vi "UHR-Fleezers Control (host) - 12.0(oscillate_test).vi"() -> ()   [LabVIEW 2014] (continued)
            n2508 = local read "Number of F/B Scans (AOD)"() -> (w4839:u16)
            n2509 = Sign(1:w4822) -> (0:w4821:dbl)
            n2510 = Compound Arithmetic op=MULTIPLY(w4822, "MCL Step Position Ratio", "MCL/AOM Scale Tweak") -> (w4826:dbl)
            n2511 = Negate(x=w4821) -> (-x=w4818:dbl)
            n2512 = Multiply(x=w4818, y="MCL Step Increment (V_int)") -> (x*y=w4820:dbl)
            n2513 = Divide(x=w4826, y="MCL X Cal (nm/V)") -> (x/y=w4832:dbl)
            n2514 = Multiply(x=32767.0 ("y"), y=w4832) -> (x*y=w4838:dbl)
            n2515 = local read "Total Counts (ticks)"() -> (w4823:u32)
            n2516 = local read "Cycles/step (AOD)"() -> (w4834:u64)
            n2517 = local read "Scan steps (AOD)"() -> (w4835:u64)
            n2518 = Divide(x=w4838, y=10.0) -> (x/y=w4831:dbl)
            n2519 = Divide(x=w4831, y="MCL Step Increment (V_int)") -> (x/y=w4829:dbl)
            n2520 = Absolute Value(x=w4829) -> (abs(x)=w4817:dbl)
            n2521 = Compound Arithmetic op=MULTIPLY(w4835, w4834, w4823) -> (w4830:u64)
            n2522 = local write "wait to reset values"(w4845) -> ()
            n2523 = local write "MCL Scanning"(w4845) -> ()
            n2524 = Divide(x=w4830, y=w4817) -> (x/y=w4827:dbl)
            "MCL Count" <- w4827
            n2525 = xnode "Read/Write Control"("FPGA VI Reference In"=w4844, "error in"=w4843, "Scan steps (MCL)"=w4817, "Number of scans (MCL)"=w4839, "Cycles per step (MCL)"=u64 1, "Scan freq.  increment (MCL)"=w4820, "1D or 2D Scan?"=w4840, "MCL Scan Axis"=w4840, "Cont. Scan (MCL)"=w4840, "MCL count"=w4827) -> ("FPGA VI Reference Out"=w4842:T22, "error out"=w4841:errorcluster)
            n2526 = xnode "Read/Write Control"("FPGA VI Reference In"=w4842, "error in"=w4841, "AI to FIFO"=w4845, "APD to FIFO"=w4845, "Start scan"=w4845, "Start scan (MCL)"=w4845) -> ("FPGA VI Reference Out"=w4847:T22, "error out"=w4846:errorcluster)
          }
        }
        "Raster Scanning..." <- TRUE ("Scanning...")
      }
    }
    n2527 = local read "Flushing P3"() -> (w3622:bool)
    n2528 = case "Keep track of when Harvard Pump 3 is done flushing" shown="True" w3622 {
      frame False {
      }
      frame True {
        n2529 = local read "Flush rate (uL/m) P3"() -> (w4005:dbl)
        n2530 = local read "DMA Update Period (s)"() -> (w3999:dbl)
        n2531 = local read "HP3 Flush Time (s)"() -> (w4013:dbl)
        n2532 = Divide(x=w4005, y=60.0) -> (x/y=w4000:dbl)
        n2533 = feedback #6(0) -> (w4011:i32)
        n2534 = Increment(x=w4011) -> (x+1=w4006:i32)
        n2535 = Divide(x=w4013, y=w3999) -> (x/y=w4007:dbl)
        n2536 = Multiply(x=w3999, y=w4000) -> (x*y=w3998:dbl)
        n2537 = Greater?(x=w4006, y=w4007) -> (0:w4010:bool)
        n2538 = feedback #7(0.0) -> (w4001:dbl)
        n2539 = Compound Arithmetic op=MULTIPLY(w3999, w4006, w4000) -> (→"P3 Flush Volume (uL)":dbl)
        n2540 = case shown="True" w4010 {
          tunnel: w4006 -> [w4014 _]
          tunnel: [w4014 0] -> w4009
          frame False {
          }
          frame True {
            w4015 = FALSE ("Flushing P3")
            n2541 = local write "Inject Pump 3"(w4015) -> ()
            n2542 = local write "Flushing P3"(w4015) -> ()
            n2543 = property on="Clear Volume P3" class="Bool (strict)"("Val(Sgnl)"=TRUE ("Value (Signaling)")) -> ()  [unwired: 2 in, 2 out]
          }
        }
        n2544 = feedback-in #6(w4009) -> ()
        n2545 = Divide(x=w4006, y=w4007) -> (x/y=→"P3 Flushing Bar":dbl)
        n2546 = Add(x=w3998, y=w4001) -> (x+y=w4002:dbl)
        "Total Volume\nFlowed P3 (uL)" <- w4002
        n2547 = feedback-in #7(w4002) -> ()
      }
    }
    n2548 = And(x="Save scans", y=w3840) -> (x .and. y?=w3879:bool)
    n2549 = local read "Flushing samp"() -> (w3615:bool)
    n2550 = case shown="True" w3615 {
      frame False {
      }
      frame True {
        n2551 = local read "DMA Update Period (s)"() -> (w3958:dbl)
        n2552 = local read "Flush rate (mL/m)"() -> (w3970:dbl)
        n2553 = local read "Samp Flush Time (s)"() -> (w3971:dbl)
        n2554 = Divide(x=w3970, y=60.0) -> (x/y=w3957:dbl)
        n2555 = feedback #8(0) -> (w3963:i32)
        n2556 = Increment(x=w3963) -> (x+1=w3962:i32)
        n2557 = Divide(x=w3971, y=w3958) -> (x/y=w3967:dbl)
        n2558 = Multiply(x=w3958, y=w3957) -> (x*y=w3956:dbl)
        n2559 = Greater?(x=w3962, y=w3967) -> (0:w3966:bool)
        n2560 = feedback #9(0.0) -> (w3959:dbl)
        n2561 = Compound Arithmetic op=MULTIPLY(w3958, w3962, w3957) -> (→"Samp Volume (uL)":dbl)
        n2562 = Divide(x=w3962, y=w3967) -> (x/y=→"Samp flush bar":dbl)
        n2563 = case shown="True" w3966 {
          tunnel: [w3972 0] -> w3965
          tunnel: w3962 -> [w3972 _]
          frame False {
          }
          frame True {
            w3975 = FALSE ("Flushing samp")
            n2564 = local write "Sample Channel\nFlow"(w3975) -> ()
            n2565 = local write "Flushing samp"(w3975) -> ()
            n2566 = property on="Clear Volume" class="Bool (strict)"("Val(Sgnl)"=TRUE) -> ()  [unwired: 2 in, 2 out]
          }
        }
        n2567 = feedback-in #8(w3965) -> ()
        n2568 = Add(x=w3956, y=w3959) -> (x+y=w3960:dbl)
        "Total Volume\nFlowed Samp (uL)" <- w3960
        n2569 = feedback-in #9(w3960) -> ()
      }
    }
    n2570 = Compound Arithmetic op=OR("Start MCL Scan", "Confocal\nImage", "Confocal\nLinescan") -> (w3838:bool)
    n2571 = And(x="Save Data (MCL)", y=w3838) -> (x .and. y?=w3878:bool)
    n2572 = case "Start MCL raster scan" shown="True" w3838 {
      tunnel: w3606 -> [w4420 w4436]
      tunnel: w3880 -> [w4419 w4435]
      tunnel: [w4420 w4431] -> w3613
      tunnel: [w4419 w4430] -> w3611
      tunnel: [FALSE w4429] -> w3864
      tunnel: "Start MCL Scan" -> [_ w4424]
      tunnel: "Confocal\nImage" -> [_ w4423]
      tunnel: "Confocal\nLinescan" -> [_ _]
      frame False {
      }
      frame True {
        w4429 = TRUE
        n2573 = case shown="True" "Restart DMA? (MCL)" {
          tunnel: [w4481 w4483] -> w4434
          tunnel: [w4480 w4482] -> w4433
          tunnel: w4436 -> [w4481 w4486]
          tunnel: w4435 -> [w4480 w4485]
          frame False {
          }
          frame True {
            n2574 = call "reset FPGA DMA.vi"("error in"=w4485, "FPGA VI Reference In"=w4486) -> ("error out"=w4482:errorcluster, "FPGA VI Reference Out"=w4483:T22)
            n2575 = local write "Overflow (data lost)"(FALSE ("Overflow (data lost)")) -> ()
          }
        }
        n2576 = case shown="False" w4424 {
          selector: w4424 -> [_ w4440]
          tunnel: w4423 -> [w4439 _]
          tunnel: [w4439 w4440] -> w4422
          frame False {
            n2577 = property on="2D or 1D Scan" class="Bool (strict)"("Val(Sgnl)"=w4439) -> ()  [unwired: 2 in, 2 out]
            n2578 = property on="Confocal\nImage" class="Bool (strict)"("Value"=FALSE ("Start Confocal Map")) -> ()  [unwired: 2 in, 2 out]
          }
          frame True {
          }
        }
        n2579 = local write "MCL Scanning"(w4429) -> ()
        n2580 = local read "AO1"() -> (w4426:dbl)
        n2581 = local read "AO2"() -> (w4425:dbl)
        n2582 = case shown="True" "Center Scan" {
          tunnel: w4434 -> [w4447 w4479]
          tunnel: w4433 -> [w4446 w4478]
          tunnel: [w4445 w4477] -> w4431
          tunnel: [w4444 w4476] -> w4430
          tunnel: [w4442 w4463] -> w4428
          tunnel: [w4441 w4462] -> w4427
          tunnel: w4426 -> [w4442 w4468]
          tunnel: w4425 -> [w4441 w4471]
          tunnel: w4422 -> [_ _]
          frame False {
            w4443 = TRUE ("AI to FIFO")
            n2583 = xnode "Read/Write Control"("FPGA VI Reference In"=w4447, "error in"=w4446, "AI to FIFO"=w4443, "APD to FIFO"=w4443, "Start scan (MCL)"=w4443) -> ("FPGA VI Reference Out"=w4445:T22, "error out"=w4444:errorcluster)
          }
          frame True {
            w4475 = TRUE ("AI to FIFO")
            n2584 = local read "Scan steps (MCL)"() -> (w4454:u64)
            n2585 = local read "Scan lines (y)"() -> (w4450:u64)
            n2586 = local read "Fast Scan Dir"() -> (w4461:bool)
            n2587 = local read "Actual MCL Inc (V)"() -> (w4451:dbl)
            n2588 = Decrement(x=w4450) -> (x-1=w4449:u64)
            n2589 = Decrement(x=w4454) -> (x-1=w4453:u64)
            n2590 = Multiply(x=w4451, y=w4449) -> (x*y=w4448:dbl)
            n2591 = Divide(x=w4448, y=2.0) -> (x/y=w4458:dbl)
            n2592 = Multiply(x=w4451, y=w4453) -> (x*y=w4452:dbl)
            n2593 = Divide(x=w4452, y=2.0) -> (x/y=w4457:dbl)
            n2594 = Select(t=w4457, s=w4461, f=w4458) -> (s? t:f=w4456:dbl)
            n2595 = Select(t=w4458, s=w4461, f=w4457) -> (s? t:f=w4460:dbl)
            n2596 = Subtract(x=w4468, y=w4460) -> (x-y=w4459:dbl)
            n2597 = Subtract(x=w4471, y=w4456) -> (x-y=w4455:dbl)
            n2598 = local read "2D or 1D Scan"() -> (w4473:bool)
            n2599 = Not(x=w4461) -> (.not. x?=w4467:bool)
            n2600 = Not(x=w4473) -> (.not. x?=w4469:bool)
            n2601 = And(x=w4461, y=w4469) -> (x .and. y?=w4470:bool)
            n2602 = And(x=w4469, y=w4467) -> (x .and. y?=w4472:bool)
            n2603 = Select(t=w4471, s=w4472, f=w4455) -> (s? t:f=w4462:dbl)
            n2604 = Select(t=w4468, s=w4470, f=w4459) -> (s? t:f=w4463:dbl)
            n2605 = call "Volt to I16.vi"("Voltage In"=w4463) -> ("I16 Voltage Out"=w4466:i16)
            n2606 = call "Volt to I16.vi"("Voltage In"=w4462) -> ("I16 Voltage Out"=w4465:i16)
            n2607 = xnode "Read/Write Control"("FPGA VI Reference In"=w4479, "error in"=w4478, "AI to FIFO"=w4475, "APD to FIFO"=w4475, "Start scan (MCL)"=w4475, "AO1"=w4466, "AO2"=w4465) -> ("FPGA VI Reference Out"=w4477:T22, "error out"=w4476:errorcluster)
          }
        }
        "Initial Y" <- w4428
        "Initial X" <- w4427
        n2608 = local write "Tab Control 6"(T3."Imaging" ("Tab Control 6")) -> ()
        "wait to reset values" <- w4429
      }
    }
    n2609 = case shown="True" "Wiggle" {
      selector: "Wiggle" -> [w3929 _]
      tunnel: w3613 -> [w3931 w3944]
      tunnel: [w3928 w3947] -> w3612
      tunnel: w3611 -> [w3930 w3942]
      tunnel: [w3927 w3946] -> w3610
      frame False {
        n2610 = xnode "Read/Write Control"("FPGA VI Reference In"=w3931, "error in"=w3930, "Wiggle trap 1"=w3929) -> ("FPGA VI Reference Out"=w3928:T22, "error out"=w3927:errorcluster)
      }
      frame True {
        w3936 = FALSE ("Abort wiggle")
        w3940 = TRUE
        n2611 = local read "Restart DMA? (AOD)"() -> (w3945:bool)
        n2612 = case shown="True" w3945 {
          tunnel: w3944 -> [w3949 w3954]
          tunnel: [w3949 w3953] -> w3943
          tunnel: w3942 -> [w3948 w3952]
          tunnel: [w3948 w3951] -> w3941
          frame False {
          }
          frame True {
            n2613 = local write "Overflow (data lost)"(FALSE) -> ()
            n2614 = call "reset FPGA DMA.vi"("error in"=w3952, "FPGA VI Reference In"=w3954) -> ("error out"=w3951:errorcluster, "FPGA VI Reference Out"=w3953:T22)
          }
        }
        n2615 = local write "Wiggle"(FALSE) -> ()
        n2616 = xnode "Read/Write Control"("FPGA VI Reference In"=w3943, "error in"=w3941, "AI to FIFO"=w3940, "APD to FIFO"=w3940, "Wiggle trap 1"="Wiggle T1", "Wiggle freq 1 (Hz)"="Wiggle freq 1 (Hz)", "Wiggle amp 1"="Wiggle amp 1 (units?)", "Abort wiggle 1"=w3936, "Wiggle trap 2"="Wiggle T2", "Abort wiggle 2"=w3936, "Wiggle freq 2 (Hz)"="Wig Freq 2 (Hz)", "Wiggle amp 2"="Wig amp 2") -> ("FPGA VI Reference Out"=w3947:T22, "error out"=w3946:errorcluster)
      }
    }
    n2617 = local read "Trap Pos Elements/DMA read"() -> (w3596:u32)
    n2618 = local read "Trap AI Elements/DMA read"() -> (w3590:u32)
    n2619 = local read "APD Elements/DMA read"() -> (w3598:u32)
    n2620 = xnode "Get APD Data"("FPGA VI Reference In"=w3612, "error in"=w3610, "Number of Elements"=w3598, "Timeout (ms)"=-1) -> ("Data"=w3774:u32[], "Elements Remaining"=→"APD FIFO Elements Remaining":u32)  [unwired: 2 out]
    n2621 = xnode "Invoke Method"("FPGA VI Reference In"=w3612, "error in"=w3610, "Number of Elements"=w3596, "Timeout (ms)"=-1) -> ("Data"=w3705:u16[], "Elements Remaining"=→"Trap Pos FIFO El Remaining":u32)  [unwired: 2 out]
    n2622 = xnode "Get Trap Data"("FPGA VI Reference In"=w3612, "error in"=w3610, "Number of Elements"=w3590, "Timeout (ms)"=-1 ("Timeout")) -> ("FPGA VI Reference Out"=w3643:T22, "error out"=w3642:errorcluster, "Data"=w3706:i16[], "Elements Remaining"=w3589:u32)
    "FIFO El. Rem." <- w3589
    n2623 = local read "Trap AI FIFO Depth"() -> (w3924:u32)
    n2624 = Subtract(x=w3924, y=w3590) -> (x-y=w3923:u32)
    n2625 = Decimate 1D Array(w3705) -> (w3594:u16[], w3592:u16[], w3593:u16[])
    n2626 = Divide(x=w3589, y=w3923) -> (x/y=w3922:dbl)
    "Buffer Status" <- w3922
    n2627 = To Unsigned Long Integer(number=w3594) -> (unsigned 32bit integer=w3704:u32[])
    n2628 = Join Numbers(hi=w3592, lo=w3593) -> ((hi.lo)=w3703:u32[])
    n2629 = Equal?(x=w3922, y=1.0) -> (x = y?=w3920:bool)
    n2630 = Join Numbers(hi=w3704, lo=w3703) -> ((hi.lo)=w3697:u64[])
    n2631 = call "IR AOM word to freq - vec.vi"("Frequency Word In (double vec)"=w3697) -> ("Frequency Out"=w3740:dbl[])
    n2632 = case "Alert buffer overflow" shown="True" w3920 {
      frame False {
      }
      frame True {
        n2633 = call <vilib>:"Beep.vi"() -> ()  [unwired: 3 in, 9 out]
        "Overflow (data lost)" <- TRUE ("Overflow (data lost)")
      }
    }
    n2634 = Decimate 1D Array(w3740) -> (w3739:dbl[], w3738:dbl[])
    n2635 = Build Array(w3739, w3738) -> (w3737:dbl[][])
    n2636 = local read "Trap Sets"() -> (w3804:u32)
    n2637 = case "Deinterlace trap data, average down PSD" shown="2" w3804 {
      tunnel: w3706 -> [w4512 w4581]
      tunnel: [w4515 w4578] -> w3797
      tunnel: [w4512 w4580] -> w3700
      tunnel: "Detector Type" -> [w4517 w4576]
      tunnel: [w4516 w4579] -> w3796
      tunnel: [w4514 w4577] -> w3897
      frame 1, Default {
        n2638 = Divide(x=w4512, y=3276.7) -> (x/y=w4513:dbl[])
        n2639 = Decimate 1D Array(w4513) -> (w4526:dbl[], w4525:dbl[], w4524:dbl[], w4523:dbl[], w4522:dbl[], w4521:dbl[], w4520:dbl[], w4519:dbl[])
        n2640 = case shown="\"IR-QPD + PSD + FB-QPD position\"" w4517 {
          tunnel: w4526 -> [w4550 w4575]
          tunnel: w4525 -> [w4549 w4574]
          tunnel: w4524 -> [w4534 w4552]
          tunnel: w4523 -> [w4535 w4562]
          tunnel: w4522 -> [w4548 w4573]
          tunnel: w4521 -> [w4547 w4572]
          tunnel: w4520 -> [w4531 w4553]
          tunnel: w4519 -> [w4530 w4551]
          tunnel: [w4529 w4559] -> w4516
          tunnel: [w4528 w4558] -> w4515
          tunnel: [w4527 w4557] -> w4514
          frame "IR-QPD + PSD + FB-QPD", Default {
            w4527 = 0  # Channel pattern
            n2641 = Divide(x=w4550, y=w4535) -> (x/y=w4537:dbl[])
            n2642 = Divide(x=w4549, y=w4535) -> (x/y=w4536:dbl[])
            n2643 = Divide(x=w4548, y=w4531) -> (x/y=w4533:dbl[])
            n2644 = Divide(x=w4547, y=w4530) -> (x/y=w4532:dbl[])
            n2645 = Build Array(w4537, w4536, w4535, w4534, w4533, w4532, w4531, w4530) -> (w4528:dbl[][])
            n2646 = Bundle("T1 Y", "T1 X", "T1 Sum", "FB Sum", "PSD Y", "PSD X", "PSD Y Sum", "PSD X Sum") -> (w4546:T47)  [unwired: 1 out]
            n2647 = Cluster To Array(cluster=w4546) -> (array=w4529:string[])
          }
          frame "IR-QPD + PSD + FB-QPD position" {
            w4557 = 3  # Channel pattern
            n2648 = Negate(x=w4553) -> (-x=w4554:dbl[])
            n2649 = Divide(x=w4575, y=w4562) -> (x/y=w4564:dbl[])
            n2650 = Divide(x=w4574, y=w4562) -> (x/y=w4563:dbl[])
            n2651 = Divide(x=w4573, y=w4553) -> (x/y=w4561:dbl[])
            n2652 = Divide(x=w4572, y=w4554) -> (x/y=w4560:dbl[])
            n2653 = Build Array(w4564, w4563, w4562, w4551, w4552, w4561, w4560, w4553) -> (w4558:dbl[][])
            n2654 = Bundle("T1 Y", "T1 X", "T1 Sum", "FB X", "FB Sum", "PSD Y", "PSD X", "PSD Y Sum") -> (w4571:T47)  [unwired: 1 out]
            n2655 = Cluster To Array(cluster=w4571) -> (array=w4559:string[])
          }
        }
      }
      frame 2 {
        n2656 = case shown="\"IR-QPD + PSD + FB-QPD XY positions\"" w4576 {
          tunnel: w4581 -> [w4643 w4710 w4779]
          tunnel: [w4594 w4706 w4724] -> w4580
          tunnel: [w4619 w4698 w4765] -> w4579
          tunnel: [w4618 w4665 w4736] -> w4578
          tunnel: [w4614 w4696 w4763] -> w4577
          frame "IR-QPD + PSD + FB-QPD", Default {
            w4614 = 1  # Channel pattern
            # "time average x2 the 4th signal and the 4 psd signals (detection laser)"
            # "deinterlace 3 signals from qpd"
            n2657 = Decimate 1D Array(w4643) -> (w4642:i16[], w4641:i16[], w4617:i16[], w4640:i16[], w4593:i16[], w4592:i16[], w4591:i16[], w4590:i16[])
            n2658 = Decimate 1D Array(w4617) -> (w4583:i16[], w4582:i16[])
            n2659 = Decimate 1D Array(w4642) -> (w4589:i16[], w4588:i16[])
            n2660 = Decimate 1D Array(w4641) -> (w4587:i16[], w4585:i16[])
            n2661 = Decimate 1D Array(w4640) -> (w4586:i16[], w4584:i16[])
            n2662 = call "downsample 1D array - double.vi"("Ave N"=2.0, "Array In"=w4593) -> ("Array Out"=w4635:dbl[])  [unwired: 1 out]
            n2663 = call "downsample 1D array - double.vi"("Ave N"=2.0, "Array In"=w4592) -> ("Array Out"=w4620:dbl[])  [unwired: 1 out]
            n2664 = call "downsample 1D array - double.vi"("Ave N"=2.0, "Array In"=w4591) -> ("Array Out"=w4634:dbl[])  [unwired: 1 out]
            n2665 = call "downsample 1D array - double.vi"("Ave N"=2.0, "Array In"=w4590) -> ("Array Out"=w4633:dbl[])  [unwired: 1 out]
            n2666 = Interleave 1D Arrays(w4589, w4587, w4586, w4588, w4585, w4584, w4583, w4582, w4635, w4620, w4634, w4633) -> (w4632:dbl[])
            n2667 = Divide(x=w4632, y=3276.7) -> (x/y=w4631:dbl[])
            n2668 = Decimate 1D Array(w4631) -> (w4630:dbl[], w4629:dbl[], w4628:dbl[], w4627:dbl[], w4626:dbl[], w4625:dbl[], w4616:dbl[], w4615:dbl[], w4624:dbl[], w4623:dbl[], w4622:dbl[], w4621:dbl[])
            n2669 = Divide(x=w4630, y=w4628) -> (x/y=w4601:dbl[])
            n2670 = Divide(x=w4629, y=w4628) -> (x/y=w4600:dbl[])
            n2671 = Divide(x=w4627, y=w4625) -> (x/y=w4599:dbl[])
            n2672 = Divide(x=w4626, y=w4625) -> (x/y=w4598:dbl[])
            n2673 = Divide(x=w4624, y=w4622) -> (x/y=w4597:dbl[])
            n2674 = Divide(x=w4623, y=w4621) -> (x/y=w4596:dbl[])
            n2675 = Build Array(w4601, w4600, w4628, w4599, w4598, w4625, w4616, w4615, w4597, w4596, w4622, w4621) -> (w4618:dbl[][])
            n2676 = Bundle("T1 Y", "T1 X", "T1 Sum", "T2 Y", "T2 X", "T2 Sum", "T1 FB Sum", "T2 FB Sum", "PSD Y", "PSD X", "PSD Y Sum", "PSD X Sum") -> (w4602:T48)  [unwired: 1 out]
            n2677 = To Word Integer(number=w4632) -> (16bit integer=w4594:i16[])
            n2678 = Cluster To Array(cluster=w4602) -> (array=w4619:string[])
          }
          frame "IR-QPD + PSD + FB-QPD X position" {
            w4696 = 2  # Channel pattern
            # "time average x2 the 3 psd signals (detection laser)"
            # "deinterlace 3 signals from qpds"
            n2679 = Decimate 1D Array(w4710) -> (w4709:i16[], w4708:i16[], w4697:i16[], w4707:i16[], w4657:i16[], w4656:i16[], w4655:i16[], w4684:i16[])
            n2680 = Decimate 1D Array(w4697) -> (w4647:i16[], w4645:i16[])
            n2681 = Decimate 1D Array(w4709) -> (w4654:i16[], w4651:i16[])
            n2682 = Decimate 1D Array(w4708) -> (w4653:i16[], w4650:i16[])
            n2683 = Decimate 1D Array(w4707) -> (w4652:i16[], w4649:i16[])
            n2684 = Decimate 1D Array(w4684) -> (w4648:i16[], w4646:i16[])
            n2685 = call "downsample 1D array - I16.vi"("Ave N"=2.0, "Array In"=w4657) -> ("Array Out"=w4662:i16[])  [unwired: 1 in]
            n2686 = call "downsample 1D array - I16.vi"("Ave N"=2.0, "Array In"=w4655) -> ("Array Out"=w4658:i16[])  [unwired: 1 in]
            n2687 = call "downsample 1D array - I16.vi"("Ave N"=2.0, "Array In"=w4656) -> ("Array Out"=w4660:i16[])  [unwired: 1 in]
            n2688 = Interleave 1D Arrays(w4654, w4653, w4652, w4651, w4650, w4649, w4648, w4647, w4646, w4645, w4662, w4660, w4658) -> (w4706:i16[])
            n2689 = Divide(x=w4706, y=3276.7) -> (x/y=w4705:dbl[])
            n2690 = Decimate 1D Array(w4705) -> (w4704:dbl[], w4703:dbl[], w4702:dbl[], w4701:dbl[], w4700:dbl[], w4699:dbl[], w4676:dbl[], w4674:dbl[], w4673:dbl[], w4671:dbl[], w4670:dbl[], w4669:dbl[], w4666:dbl[])
            n2691 = Negate(x=w4666) -> (-x=w4664:dbl[])
            n2692 = Divide(x=w4670, y=w4666) -> (x/y=w4668:dbl[])
            n2693 = Divide(x=w4669, y=w4664) -> (x/y=w4667:dbl[])
            n2694 = Divide(x=w4704, y=w4702) -> (x/y=w4688:dbl[])
            n2695 = Divide(x=w4703, y=w4702) -> (x/y=w4687:dbl[])
            n2696 = Divide(x=w4701, y=w4699) -> (x/y=w4686:dbl[])
            n2697 = Divide(x=w4700, y=w4699) -> (x/y=w4685:dbl[])
            n2698 = Divide(x=w4676, y=w4674) -> (x/y=w4675:dbl[])
            n2699 = Divide(x=w4673, y=w4671) -> (x/y=w4672:dbl[])
            n2700 = Build Array(w4688, w4687, w4702, w4686, w4685, w4699, w4675, w4674, w4672, w4671, w4668, w4667, w4666) -> (w4665:dbl[][])
            n2701 = Bundle("T1 Y", "T1 X", "T1 Sum", "T2 Y", "T2 X", "T2 Sum", "T1 FB X", "T1 FB Sum", "T2 FB X", "T2 FB Sum", "PSD Y", "PSD X", "PSD Y Sum") -> (w4689:T49)  [unwired: 1 out]
            n2702 = Cluster To Array(cluster=w4689) -> (array=w4698:string[])
          }
          frame "IR-QPD + PSD + FB-QPD XY positions" {
            w4763 = 4  # Channel pattern
            # "time average x2 the 3 psd signals (detection laser)"
            # "deinterlace 3 signals from qpds"
            n2703 = Decimate 1D Array(w4779) -> (w4778:i16[], w4777:i16[], w4764:i16[], w4776:i16[], w4734:i16[], w4752:i16[])  [unwired: 2 out]
            n2704 = Decimate 1D Array "Feedback Sum"(w4764) -> (w4715:i16[], w4712:i16[])
            n2705 = Decimate 1D Array "QPD Y"(w4778) -> (w4723:i16[], w4720:i16[])
            n2706 = Decimate 1D Array "QPD X"(w4777) -> (w4722:i16[], w4719:i16[])
            n2707 = Decimate 1D Array "Feedback Y"(w4734) -> (w4717:i16[], w4714:i16[])
            n2708 = Decimate 1D Array "QPD Sum"(w4776) -> (w4721:i16[], w4718:i16[])
            n2709 = Decimate 1D Array "Feedback X"(w4752) -> (w4716:i16[], w4713:i16[])
            n2710 = call "downsample 1D array - double.vi"("Ave N"=2.0) -> ("Array Out"=w4751:dbl[])  [unwired: 1 in, 1 out]
            n2711 = call "downsample 1D array - double.vi"("Ave N"=2.0) -> ("Array Out"=w4750:dbl[])  [unwired: 1 in, 1 out]
            n2712 = Interleave 1D Arrays(w4723, w4722, w4721, w4720, w4719, w4718, w4717, w4716, w4715, w4714, w4713, w4712, w4751, w4750) -> (w4773:dbl[])
            n2713 = Divide(x=w4773, y=3276.7) -> (x/y=w4772:dbl[])
            n2714 = Decimate 1D Array(w4772) -> (w4771:dbl[], w4770:dbl[], w4769:dbl[], w4768:dbl[], w4767:dbl[], w4766:dbl[], w4731:dbl[], w4743:dbl[], w4729:dbl[], w4730:dbl[], w4741:dbl[], w4727:dbl[], w4739:dbl[], w4737:dbl[])
            n2715 = Negate(x=w4737) -> (-x=w4735:dbl[])
            n2716 = Divide(x=w4739, y=w4735) -> (x/y=w4738:dbl[])
            n2717 = Divide(x=w4730, y=w4727) -> (x/y=w4726:dbl[])
            n2718 = Divide(x=w4731, y=w4729) -> (x/y=w4728:dbl[])
            n2719 = Divide(x=w4771, y=w4769) -> (x/y=w4756:dbl[])
            n2720 = Divide(x=w4770, y=w4769) -> (x/y=w4755:dbl[])
            n2721 = Divide(x=w4768, y=w4766) -> (x/y=w4754:dbl[])
            n2722 = Divide(x=w4767, y=w4766) -> (x/y=w4753:dbl[])
            n2723 = Divide(x=w4743, y=w4729) -> (x/y=w4742:dbl[])
            n2724 = Divide(x=w4741, y=w4727) -> (x/y=w4740:dbl[])
            n2725 = Build Array(w4756, w4755, w4769, w4754, w4753, w4766, w4728, w4742, w4729, w4726, w4740, w4727, w4738, w4737) -> (w4736:dbl[][])
            n2726 = Bundle("T1 Y", "T1 X", "T1 Sum", "T2 Y", "T2 X", "T2 Sum", "T1 FB Y", "T1 FB X", "T1 FB Sum", "T2 FB Y", "T2 FB X", "T2 FB Sum", "PSD X", "PSD Y Sum") -> (w4725:T50)  [unwired: 1 out]
            n2727 = To Word Integer(number=w4773) -> (16bit integer=w4724:i16[])
            n2728 = Cluster To Array(cluster=w4725) -> (array=w4765:string[])
          }
        }
      }
    }
    "AI labels" <- w3796
    n2729 = Decimate 1D Array(w3774) -> (w3584:u32[], w3585:u32[])
    n2730 = local read "DMA Update Period (s)"() -> (w3805:dbl)
    n2731 = Build Array(w3584, w3585) -> (w3588:u32[][])
    n2732 = local read "Data Period (s)"() -> (w3659:dbl)
    n2733 = local read "BD 1 Frequency 2 (MHz)"() -> (w3692:dbl)
    n2734 = local read "BD 1 Frequency 1 (MHz)"() -> (w3693:dbl)
    n2735 = Decimate 1D Array(w3700) -> (w3720:i16[], w3719:i16[], w3717:i16[], w3716:i16[])  [unwired: 9 out]
    n2736 = To Double Precision Float(number=w3588) -> (double precision float=w3862:dbl[][])
    n2737 = local read "APD Integration Time (s)"() -> (w3756:dbl)
    n2738 = Multiply(x=w3659, y="Trap Pos. Disp. Downsample") -> (x*y=w3657:dbl)
    n2739 = Divide(x=w3720, y=w3719) -> (x/y=w3721:dbl[])
    n2740 = Divide(x=w3717, y=w3716) -> (x/y=w3718:dbl[])
    n2741 = feedback #10(0.0) -> (w3734:dbl)
    n2742 = Add(x=w3805, y=w3734) -> (x+y=w3899:dbl)
    n2743 = feedback-in #10(w3899) -> ()
    n2744 = local read "AOM X Cal (nm/MHz)"() -> (w3690:dbl)
    n2745 = To Time Stamp(1:w3734) -> (0:w3733:timestamp)
    n2746 = Split 1D Array(array=w3721, index="N El. to Ave.") -> (second subarray=w3724:dbl[])  [unwired: 1 out]
    n2747 = Split 1D Array(array=w3718, index="N El. to Ave.") -> (second subarray=w3723:dbl[])  [unwired: 1 out]
    n2748 = Multiply(x=w3659, y="Trap Disp. Downsample") -> (x*y=w3735:dbl)
    "Display Period (s)" <- w3735
    n2749 = for "Trap AI" {
      tunnel: [w4511] -> w3893 mode=indexing
      tunnel: w3733 -> [w4501]
      tunnel: "Trap Disp. Downsample" -> [w4509]
      tunnel: w3797 -> [w4507] mode=indexing
      tunnel: w3659 -> [w4506]
      tunnel: w3796 -> [w4505] mode=indexing
      tunnel: w3732 -> [w4504]
      tunnel: [w4503] -> w3766 mode=indexing
      tunnel: w3735 -> [w4502]
      workers-P: _ -> [_]
      n2750 = Bundle By Name("Y"=w4507, "dt"=w4506) -> (w4508:waveform(dbl))  [unwired: 1 out]
      n2751 = Set Waveform Attribute(5:w4505, 6:w4504, 7:w4508) -> (3:w4503:waveform(dbl))  [unwired: 1 in, 2 out]
      n2752 = call "downsample 1D array - double.vi"("Ave N"=w4509, "Array In"=w4507) -> ("Array Out"=w4510:dbl[])  [unwired: 1 out]
      n2753 = Bundle By Name(cluster=w4503, "t0"=w4501, "Y"=w4510, "dt"=w4502) -> (w4511:waveform(dbl))
    }
    n2754 = Bundle("BD 1 Frequency 1 (MHz)"=w3693, "BD 1 Frequency 2 (MHz)"=w3692) -> (w3694:T51)  [unwired: 1 out]
    n2755 = call-poly <vilib>:"Mean.vi"("X"=w3723) -> ("mean"=w3711:dbl)  [unwired: 1 out]
    n2756 = call-poly <vilib>:"Mean.vi"("X"=w3724) -> ("mean"=w3712:dbl)  [unwired: 1 out]
    n2757 = Reciprocal(x=w3735) -> (1/x=→"Trap Disp. Freq. (Hz)":dbl)
    n2758 = Cluster To Array(cluster=w3694) -> (array=w3691:dbl[])
    n2759 = local read "Trap X AI1 (DMA)"() -> (w3722:T13)
    n2760 = local read "Data points/scans (MCL)"() -> (w3873:dbl)
    n2761 = To Fixed-Point(number=w3711) -> (fixed-point=w3709:fxp<+/-,16,1>)  [unwired: 1 in]
    n2762 = To Fixed-Point(number=w3712) -> (fixed-point=w3710:fxp<+/-,16,1>)  [unwired: 1 in]
    n2763 = Bundle("Trap 1 Pos.", "Trap 2 Pos.") -> (w3731:cluster{string, string})  [unwired: 1 out]
    n2764 = Bundle By Name(cluster=w3722, "Set 1"=w3710, "Set 2"=w3709) -> (→"Trap X AI1 (DMA)":T13)
    n2765 = Cluster To Array(cluster=w3731) -> (array=w3728:string[])
    n2766 = Bundle("APD 1", "APD 2") -> (w3892:cluster{string, string})  [unwired: 1 out]
    n2767 = Select(t=-1.0, s="Negate Y Axis", f=1.0) -> (s? t:f=w3676:dbl)
    n2768 = for "Trap Position" {
      tunnel: w3737 -> [w4143] mode=indexing
      tunnel: "Trap Pos. Disp. Downsample" -> [w4142]
      tunnel: w3657 -> [w4140]
      tunnel: w3733 -> [w4139]
      tunnel: w3732 -> [w4137]
      tunnel: w3728 -> [w4136] mode=indexing
      tunnel: [w4135] -> w3646 mode=indexing
      tunnel: w3691 -> [w4133] mode=indexing
      tunnel: w3690 -> [w4131]
      tunnel: w3676 -> [w4130]
      n2769 = call "downsample 1D array - double.vi"("Ave N"=w4142, "Array In"=w4143) -> ("Array Out"=w4141:dbl[])  [unwired: 1 out]
      n2770 = Subtract(x=w4141, y=w4133) -> (x-y=w4134:dbl[])
      n2771 = Multiply(x=w4131, y=w4134) -> (x*y=w4132:dbl[])
      n2772 = Multiply(x=w4130, y=w4132) -> (x*y=w4129:dbl[])
      n2773 = Bundle By Name("Y"=w4129, "dt"=w4140, "t0"=w4139) -> (w4138:waveform(dbl))  [unwired: 1 out]
      n2774 = Set Waveform Attribute(5:w4136, 6:w4137, 7:w4138) -> (3:w4135:waveform(dbl))  [unwired: 1 in, 2 out]
    }
    n2775 = Cluster To Array(cluster=w3892) -> (array=w3889:string[])
    n2776 = for "APD" {
      tunnel: w3862 -> [w4487] mode=indexing
      tunnel: w3756 -> [w4498]
      tunnel: [w4494] -> w3762 mode=indexing
      tunnel: "APD Disp. Scale" -> [w4495]
      tunnel: w3732 -> [w4493]
      tunnel: w3889 -> [w4492] mode=indexing
      tunnel: "APD Disp. Downsample" -> [w4489]
      tunnel: [w4491] -> w3888
      workers-P: _ -> [_]
      tunnel: w3733 -> [w4488]
      n2777 = call "integrate 1D array interval - double.vi"("Ave N"=w4489, "Array In"=w4487) -> ("Array Out"=w4490:dbl[])  [unwired: 1 out]
      n2778 = Multiply(x=w4498, y=w4489) -> (x*y=w4491:dbl)
      n2779 = Divide(x=w4490, y=w4495) -> (x/y=w4496:dbl[])
      n2780 = Bundle By Name("t0"=w4488, "Y"=w4496, "dt"=w4491) -> (w4497:waveform(dbl))  [unwired: 1 out]
      n2781 = Set Waveform Attribute(5:w4492, 6:w4493, 7:w4497) -> (3:w4494:waveform(dbl))  [unwired: 1 in, 2 out]
    }
    "APD Display Period (s)" <- w3888
    n2782 = Reciprocal(x=w3888) -> (1/x=→"APD Display Freq. (Hz)":dbl)
    n2783 = local read "Display Period (s)"() -> (w3783:dbl)
    n2784 = Increment(x=w3873) -> (x+1=w3874:dbl)
    n2785 = To Double Precision Float(number=w3584) -> (double precision float=w3794:dbl[])
    n2786 = Index Array(array=w3646, index=0) -> (element=w3650:waveform(dbl))
    n2787 = Index Array(array=w3646, index=1) -> (element=w3645:waveform(dbl))
    n2788 = feedback #11(w3874) -> (w3877:dbl)
    n2789 = Select(t=0, s=w3864, f=w3877) -> (s? t:f=w3870:dbl)
    n2790 = Array Size(array=w3794) -> (size(s)=w3876:i32)
    n2791 = Add(x=w3876, y=w3870) -> (x+y=w3871:dbl)
    n2792 = Unbundle By Name(w3650) -> ("Y"=w3651:dbl[])
    n2793 = feedback #12(w3584) -> (w3861:u32[])
    n2794 = Build Array (concatenate)(w3861, w3584) -> (w3858:u32[])
    n2795 = feedback #13(w3585) -> (w3761:u32[])
    n2796 = Divide(x="Bead Sep. Int. Time (s)", y=w3783) -> (x/y=w3686:dbl)
    n2797 = Build Array (concatenate)(w3761, w3585) -> (w3760:u32[])
    n2798 = Add(x=w3651, y="FB Trap Pos Offset") -> (x+y=w3649:dbl[])
    "T1 x pos data" <- w3649
    n2799 = Greater?(x=w3871, y=w3873) -> (0:w3872:bool)
    n2800 = feedback #14(w3649) -> (w3688:dbl[])
    n2801 = Build Array (concatenate)(w3649, w3688) -> (w3687:dbl[])
    n2802 = Bundle By Name(cluster=w3650, "Y"=w3649) -> (w3648:waveform(dbl))
    n2803 = Select(t=w3870, s=w3872, f=w3871) -> (s? t:f=w3869:dbl)
    n2804 = feedback-in #11(w3869) -> ()
    n2805 = Array Size(array=w3858) -> (size(s)=w3855:i32)
    n2806 = Array Size(array=w3584) -> (size(s)=w3857:i32)
    n2807 = local read "MCL Scanning"() -> (w3867:bool)
    n2808 = local read "APD Integration Time (s)"() -> (w3769:dbl)
    n2809 = Bundle(w3648, w3645) -> (w3644:cluster{waveform(dbl), waveform(dbl)})  [unwired: 1 out]
    n2810 = Build Array (concatenate)(w3762, w3893) -> (w3764:waveform(dbl)[])
    "All Signals" <- w3764
    n2811 = Split 1D Array(array=w3687, index=w3686) -> (first subarray=w3680:dbl[])  [unwired: 1 out]
    n2812 = feedback-in #14(w3680) -> ()
    n2813 = Multiply(x=w3857, y="APD Ave N") -> (x*y=w3856:dbl)
    n2814 = Greater?(x=w3855, y=w3856) -> (0:w3859:bool)
    n2815 = Not(x=w3872) -> (.not. x?=w3866:bool)
    n2816 = Cluster To Array(cluster=w3644) -> (array=w3620:waveform(dbl)[])
    "Trap Positions" <- w3620
    n2817 = To Double Precision Float(number=w3585) -> (double precision float=w3743:dbl[])
    n2818 = call-poly <vilib>:"Mean.vi"("X"=w3680) -> ("mean"=w3679:dbl)  [unwired: 1 out]
    "Mean T1 Position (nm)" <- w3679
    n2819 = Subtract(x=w3680, y=w3679) -> (x-y=w3685:dbl[])
    n2820 = Square(x=w3685) -> (x^2=w3684:dbl[])
    n2821 = And(x=w3866, y=w3867) -> (x .and. y?=w3868:bool)
    n2822 = call-poly <vilib>:"Mean.vi"("X"=w3684) -> ("mean"=w3683:dbl)  [unwired: 1 out]
    n2823 = case shown="True" w3859 {
      tunnel: w3858 -> [w4270 w4272]
      tunnel: [w4270 w4276] -> w3586
      tunnel: w3856 -> [_ w4274]
      tunnel: w3855 -> [_ w4277]
      tunnel: w3760 -> [w4269 w4271]
      tunnel: [w4269 w4273] -> w3587
      frame False {
      }
      frame True {
        n2824 = Subtract(x=w4277, y=w4274) -> (x-y=w4275:dbl)
        n2825 = Array Subset(array=w4272, index=w4275, length=w4274) -> (w4276:u32[])
        n2826 = Array Subset(array=w4271, index=w4275, length=w4274) -> (w4273:u32[])
      }
    }
    n2827 = feedback-in #12(w3586) -> ()
    n2828 = feedback-in #13(w3587) -> ()
    n2829 = Square Root(x=w3683) -> (sqrt(x)=w3682:dbl)
    n2830 = Or(x=w3868, y=w3864) -> (x .or. y?=w3865:bool)
    n2831 = Equal?(x="Tab Control 6", y=T41."High Res Display") -> (x = y?=w3800:bool)
    n2832 = Multiply(x="APD Disp. Scale", y=w3762) -> (x*y=w3771:waveform(dbl)[])
    n2833 = Multiply(x=10.0, y=w3682) -> (x*y=→"Trap 1 Position RMS (A)":dbl)
    n2834 = Multiply(x="APD Disp. Downsample", y=w3769) -> (x*y=w3767:dbl)
    n2835 = Divide(x=w3771, y=w3767) -> (x/y=w3741:waveform(dbl)[])
    n2836 = case "For displaying the high resolution display (no downsampling)" shown="True" w3800 {
      tunnel: w3766 -> [_ w4168]
      frame False {
      }
      frame True {
        n2837 = Index Array(array=w4168, index="High Res. Display") -> (element=w4169:waveform(dbl))
        n2838 = call <vilib>:"Std Deviation and Variance.vi"("X"=w4169) -> ("mean"=w4176:dbl, "standard deviation"=w4181:dbl)  [unwired: 1 in, 1 out]
        "Mean Intensity" <- w4176
        "Sigma" <- w4181
        n2839 = Subtract(x=w4169, y=w4176) -> (x-y=w4175:waveform(dbl))
        n2840 = Select(t=w4175, s="Subtract mean", f=w4169) -> (s? t:f=→"1 Channel":waveform(dbl))
        n2841 = Divide(x=w4181, y=w4176) -> (x/y=→"Sigma/Mean":dbl)
        n2842 = feedback #15(1) -> (w4170:i32)
        n2843 = Greater Or Equal?(x=w4170, y="Slow mean N ave.") -> (x >= y?=w4183:bool)
        n2844 = Increment(x=w4170) -> (x+1=w4185:i32)
        n2845 = Select(t=1, s=w4183, f=w4185) -> (s? t:f=w4172:i32)
        n2846 = feedback-in #15(w4172) -> ()
        n2847 = feedback #16() -> (w4173:waveform(dbl))  [unwired: 1 out]
        n2848 = case shown="Default" w4170 {
          tunnel: [w4188 w4191] -> w4174
          tunnel: w4173 -> [w4190 _]
          tunnel: w4169 -> [w4189 w4191]
          frame Default {
            n2849 = call-poly <vilib>:"Append Waveforms.vi"("waveform B"=w4189, "waveform A"=w4190) -> ("waveform out"=w4188:waveform(dbl))  [unwired: 1 in, 8 out]
          }
          frame 1 {
          }
        }
        n2850 = feedback-in #16(w4174) -> ()
        n2851 = case shown="True" w4183 {
          tunnel: w4174 -> [_ w4187]
          frame False {
          }
          frame True {
            n2852 = call-poly <vilib>:"Mean.vi"("X"=w4187) -> ("mean"=→"Slow mean":dbl)  [unwired: 1 out]
          }
        }
      }
    }
    n2853 = Index Array(array=w3741, index=0) -> (element=w3750:waveform(dbl))
    n2854 = Index Array(array=w3741, index=1) -> (element=w3748:waveform(dbl))
    n2855 = case "For computing FFTs for display" shown="True" "Compute FFT" {
      tunnel: w3766 -> [_ w4882]
      frame False {
      }
      frame True {
        n2856 = Build Array("FFT 1 Choice 1", "FFT 1 Choice 2", "FFT 2 Choice 1", "FFT 2 Choice 2") -> (w4875:u16[])
        n2857 = Array Size(array=w4882) -> (size(s)=w4881:i32)
        n2858 = feedback-in #17(w4875) -> ()
        n2859 = feedback #17(u16[] [100, 100, 100, 100]) -> (w4876:u16[])
        n2860 = feedback-in #18("# Spectra to Ave.") -> ()
        n2861 = feedback #18("# Spectra to Ave.") -> (w4873:dbl)
        n2862 = Not Equal?(x="# Spectra to Ave.", y=w4873) -> (x != y?=w4872:bool)
        n2863 = Not Equal?(x=w4875, y=w4876) -> (x != y?=w4874:bool)
        n2864 = feedback #19(1.0) -> (w4859:dbl)
        n2865 = Compound Arithmetic op=OR("Reset FFT", w4874, w4872) -> (w4857:bool)
        n2866 = Select(t=1.0, s=w4857, f=w4859) -> (s? t:f=w4861:dbl)
        n2867 = Greater?(x=w4861, y="# Spectra to Ave.") -> (0:w4880:bool)
        n2868 = Increment(x=w4861) -> (x+1=w4860:dbl)
        n2869 = feedback-in #19(w4860) -> ()
        n2870 = local read "DMA Update Period (s)"() -> (w4855:dbl)
        n2871 = Multiply(x="# Spectra to Ave.", y=w4855) -> (x*y=→"Ave. Time (s)":dbl)
        n2872 = Build Array(cluster{"f0":dbl, "df":dbl, "magnitude":dbl[]} {"f0"=0.0, "df"=0.0, "magnitude"=[]} ("PSD")) -> (w4864:cluster{"f0":dbl, "df":dbl, "magnitude":dbl[]}[])
        n2873 = Build Array(w4864, w4864, w4864, w4864) -> (w4866:T52)
        n2874 = feedback #20(w4866) -> (w4871:T52)
        n2875 = for {
          N: 4 -> [_]
          tunnel: w4875 -> [w4904] mode=indexing
          tunnel: w4882 -> [w4905]
          tunnel: w4881 -> [w4907]
          tunnel: w4857 -> [w4900]
          tunnel: w4880 -> [w4899]
          tunnel: "# Spectra to Ave." -> [w4898]
          tunnel: [w4897] -> w4870 mode=indexing
          tunnel: w4871 -> [w4902] mode=indexing
          tunnel: [w4901] -> w4858 mode=indexing
          tunnel: w4861 -> [w4896]
          n2876 = Less?(x=w4904, y=w4907) -> (x < y?=w4906:bool)
          n2877 = Index Array(array=w4905, index=w4904) -> (element=w4903:waveform(dbl))
          n2878 = case shown="True" w4906 {
            tunnel: w4903 -> [_ w4924]
            tunnel: w4902 -> [w4909 w4922]
            tunnel: [w4909 w4910] -> w4901
            tunnel: w4900 -> [_ w4921]
            tunnel: w4899 -> [_ w4914]
            tunnel: w4898 -> [_ w4913]
            tunnel: [cluster{"f0":dbl, "df":dbl, "magnitude":dbl[]} {"f0"=0.0, "df"=0.0, "magnitude"=[]} ("PSD") w4915] -> w4897
            tunnel: w4896 -> [_ w4912]
            frame False {
            }
            frame True {
              n2879 = call <vilib>:"Std Deviation and Variance.vi"("X"=w4924) -> ("mean"=w4925:dbl)  [unwired: 1 in, 2 out]
              n2880 = Subtract(x=w4924, y=w4925) -> (x-y=w4923:waveform(dbl))
              n2881 = xnode "Spectral Measurements"("Signals"=w4923) -> ("PSD"=w4917:cluster{"f0":dbl, "df":dbl, "magnitude":dbl[]})  [unwired: 1 in, 1 out]
              n2882 = case shown="False" w4921 {
                tunnel: w4922 -> [w4934 _]
                tunnel: [w4930 w4939] -> w4910
                tunnel: w4917 -> [w4933 w4940]
                tunnel: w4914 -> [w4932 _]
                frame False {
                  n2883 = Build Array (concatenate)(w4934, w4933) -> (w4931:cluster{"f0":dbl, "df":dbl, "magnitude":dbl[]}[])
                  n2884 = case shown="True" w4932 {
                    tunnel: w4931 -> [w4935 w4938]
                    tunnel: [w4935 w4936] -> w4930
                    frame False {
                    }
                    frame True {
                      n2885 = Delete From Array(array=w4938, index=0) -> (array with subset deleted=w4936:cluster{"f0":dbl, "df":dbl, "magnitude":dbl[]}[])  [unwired: 1 in, 1 out]
                    }
                  }
                }
                frame True {
                  n2886 = Build Array(w4940) -> (w4939:cluster{"f0":dbl, "df":dbl, "magnitude":dbl[]}[])
                }
              }
              n2887 = for {
                tunnel: w4910 -> [w4929] mode=indexing
                tunnel: [w4928] -> w4920 mode=indexing
                workers-P: _ -> [_]
                n2888 = Unbundle By Name(w4929) -> ("magnitude"=w4928:dbl[])
              }
              n2889 = Transpose 2D Array(2D array=w4920) -> (transposed array=w4919:dbl[][])
              n2890 = for {
                tunnel: w4919 -> [w4927] mode=indexing
                tunnel: [w4926] -> w4918 mode=indexing
                workers-P: _ -> [_]
                n2891 = Add Array Elements(numeric array=w4927) -> (sum=w4926:dbl)
              }
              n2892 = Select(t=w4913, s=w4914, f=w4912) -> (s? t:f=w4911:dbl)
              n2893 = Divide(x=w4918, y=w4911) -> (x/y=w4916:dbl[])
              n2894 = Bundle By Name(cluster=w4917, "magnitude"=w4916) -> (w4915:cluster{"f0":dbl, "df":dbl, "magnitude":dbl[]})
            }
          }
        }
        n2895 = case shown="True" w4857 {
          tunnel: w4858 -> [w4889 w4895]
          tunnel: [w4889 w4890] -> w4856
          frame False {
          }
          frame True {
            n2896 = Array Subset(array=w4895, index (row)=0 ("index"), length (row)=4 ("length"), index (col)=0 ("index"), length (col)=1 ("length")) -> (w4890:T52)
          }
        }
        n2897 = feedback-in #20(w4856) -> ()
        n2898 = Split 1D Array(array=w4870, index=2) -> (first subarray=→"FFT 1":cluster{"f0":dbl, "df":dbl, "magnitude":dbl[]}[], second subarray=→"FFT 2":cluster{"f0":dbl, "df":dbl, "magnitude":dbl[]}[])
      }
    }
    n2899 = case "For plotting results of scanning MCL" shown="True" w3865 {
      tunnel: w3864 -> [_ w4310]
      tunnel: w3794 -> [_ w4406]
      tunnel: w3873 -> [_ _]
      tunnel: w3766 -> [_ w4380]
      tunnel: w3743 -> [_ w4311]
      tunnel: w3742 -> [_ w4284]
      frame False {
      }
      frame True {
        w4291 = u32 0 items=["Horizontal", "Vertical", "Central", "1st Diagonal", "2nd Diagonal"] ("Type of Symmetry")
        w4319 = u32 0 items=["Horizontal", "Vertical", "Central", "1st Diagonal", "2nd Diagonal"] ("Type of Symmetry")
        w4322 = u32 0 items=["Horizontal", "Vertical", "Central", "1st Diagonal", "2nd Diagonal"] ("Type of Symmetry")
        w4351 = u32 0 items=["Horizontal", "Vertical", "Central", "1st Diagonal", "2nd Diagonal"] ("Type of Symmetry")
        n2900 = Index Array(array=w4380, index=10) -> (element=w4386:waveform(dbl))
        n2901 = Index Array(array=w4380, index=11) -> (element=w4383:waveform(dbl))
        n2902 = local read "Cycles/step (MCL)"() -> (w4336:u64)
        n2903 = Index Array(array=w4380, index="Channel") -> (element=w4382:waveform(dbl))
        n2904 = Unbundle(w4284) -> ("New Image"=w4283:T2, "New Image"=w4282:T2, "New Image"=w4281:T2, "New Image"=w4280:T2)
        n2905 = Unbundle By Name(w4386) -> ("Y"=w4338:dbl[])
        n2906 = Unbundle By Name(w4383) -> ("Y"=w4340:dbl[])
        n2907 = Unbundle By Name(w4382) -> ("Y"=w4345:dbl[])
        n2908 = call "downsample 1D array - double.vi"("Ave N"=w4336, "Array In"=w4338) -> ("Array Out"=w4337:dbl[])  [unwired: 1 out]
        n2909 = call "downsample 1D array - double.vi"("Ave N"=w4336, "Array In"=w4340) -> ("Array Out"=w4339:dbl[])  [unwired: 1 out]
        n2910 = call "downsample 1D array - double.vi"("Ave N"=w4336, "Array In"=w4345) -> ("Array Out"=w4344:dbl[])  [unwired: 1 out]
        n2911 = feedback #21(w4406) -> (w4407:dbl[])
        n2912 = Build Array (concatenate)(w4407, w4406) -> (w4388:dbl[])
        n2913 = feedback #22(w4311) -> (w4313:dbl[])
        n2914 = Build Array (concatenate)(w4313, w4311) -> (w4312:dbl[])
        n2915 = local read "Scan steps (MCL)"() -> (w4293:u64)
        n2916 = Select(t=w4406, s=w4310, f=w4388) -> (s? t:f=w4392:dbl[])
        n2917 = feedback-in #21(w4392) -> ()
        n2918 = Select(t=w4311, s=w4310, f=w4312) -> (s? t:f=w4294:dbl[])
        n2919 = feedback-in #22(w4294) -> ()
        n2920 = local read "Scan lines (y)"() -> (w4279:u64)
        n2921 = local read "N APD Samp/step"() -> (w4295:dbl)
        n2922 = feedback #23(w4337) -> (w4394:dbl[])
        n2923 = Build Array (concatenate)(w4394, w4337) -> (w4385:dbl[])
        n2924 = feedback #24(w4344) -> (w4404:dbl[])
        n2925 = Build Array (concatenate)(w4404, w4344) -> (w4403:dbl[])
        n2926 = feedback #25(w4339) -> (w4396:dbl[])
        n2927 = Build Array (concatenate)(w4396, w4339) -> (w4397:dbl[])
        n2928 = Select(t=w4337, s=w4310, f=w4385) -> (s? t:f=w4341:dbl[])
        n2929 = feedback-in #23(w4341) -> ()
        n2930 = Select(t=w4344, s=w4310, f=w4403) -> (s? t:f=w4343:dbl[])
        n2931 = feedback-in #24(w4343) -> ()
        n2932 = Select(t=w4339, s=w4310, f=w4397) -> (s? t:f=w4342:dbl[])
        n2933 = feedback-in #25(w4342) -> ()
        n2934 = Multiply(x=w4293, y=u64 2) -> (x*y=w4278:u64)
        n2935 = call "integrate 1D array interval - double.vi"("Ave N"=w4295, "Array In"=w4294) -> ("Array Out"=w4306:dbl[])  [unwired: 1 out]
        n2936 = call "integrate 1D array interval - double.vi"("Ave N"=w4295, "Array In"=w4392) -> ("Array Out"=w4391:dbl[])  [unwired: 1 out]
        n2937 = Array Size(array=w4306) -> (size(s)=w4307:i32)
        n2938 = Array Size(array=w4391) -> (size(s)=w4393:i32)
        n2939 = Multiply(x=w4279, y=w4278) -> (x*y=w4309:u64)
        n2940 = Multiply(x=w4279, y=w4278) -> (x*y=w4401:u64)
        n2941 = call-poly <vilib>:"Mean.vi"("X"=w4341) -> ("mean"=w4325:dbl)  [unwired: 1 out]
        n2942 = Subtract(x=w4309, y=w4307) -> (x-y=w4300:u64)
        n2943 = call-poly <vilib>:"Mean.vi"("X"=w4343) -> ("mean"=w4330:dbl)  [unwired: 1 out]
        n2944 = call-poly <vilib>:"Mean.vi"("X"=w4342) -> ("mean"=w4328:dbl)  [unwired: 1 out]
        n2945 = call-poly <vilib>:"Mean.vi"("X"=w4306) -> ("mean"=w4297:dbl)  [unwired: 1 out]
        n2946 = Subtract(x=w4401, y=w4393) -> (x-y=w4335:u64)
        n2947 = call-poly <vilib>:"Mean.vi"("X"=w4391) -> ("mean"=w4332:dbl)  [unwired: 1 out]
        n2948 = Initialize Array(1.0 ("element"), w4300) -> (w4296:dbl[])
        n2949 = Initialize Array(1.0 ("element"), w4335) -> (w4326:dbl[])
        n2950 = Multiply(x=w4296, y=w4297) -> (x*y=w4298:dbl[])
        n2951 = Multiply(x=w4326, y=w4328) -> (x*y=w4329:dbl[])
        n2952 = Multiply(x=w4326, y=w4330) -> (x*y=w4331:dbl[])
        n2953 = Multiply(x=w4326, y=w4325) -> (x*y=w4327:dbl[])
        n2954 = Multiply(x=w4326, y=w4332) -> (x*y=w4333:dbl[])
        n2955 = Build Array (concatenate)(w4341, w4327) -> (w4395:dbl[])
        n2956 = Build Array (concatenate)(w4343, w4331) -> (w4399:dbl[])
        n2957 = Build Array (concatenate)(w4342, w4329) -> (w4398:dbl[])
        n2958 = Build Array (concatenate)(w4306, w4298) -> (w4308:dbl[])
        n2959 = Build Array (concatenate)(w4391, w4333) -> (w4400:dbl[])
        n2960 = Reshape Array(w4395, w4279, w4278) -> (w4361:dbl[][])
        n2961 = Reshape Array(w4308, w4279, w4278) -> (w4304:dbl[][])
        n2962 = Reshape Array(w4399, w4279, w4278) -> (w4353:dbl[][])
        n2963 = Reshape Array(w4398, w4279, w4278) -> (w4368:dbl[][])
        n2964 = Reshape Array(w4400, w4279, w4278) -> (w4378:dbl[][])
        n2965 = Array Subset(array=w4368, index (col)=0 ("index"), length (col)=w4293) -> (w4373:dbl[][])  [unwired: 2 in]
        n2966 = Array Subset(array=w4368, index (col)=w4293) -> (w4371:dbl[][])  [unwired: 3 in]
        n2967 = Array Subset(array=w4353, index (col)=0 ("index"), length (col)=w4293) -> (w4359:dbl[][])  [unwired: 2 in]
        n2968 = Array Subset(array=w4353, index (col)=w4293) -> (w4357:dbl[][])  [unwired: 3 in]
        n2969 = Array Subset(array=w4304, index (col)=0 ("index"), length (col)=w4293) -> (w4303:dbl[][])  [unwired: 2 in]
        n2970 = Array Subset(array=w4304, index (col)=w4293) -> (w4301:dbl[][])  [unwired: 3 in]
        n2971 = Array Subset(array=w4378, index (col)=0 ("index"), length (col)=w4293) -> (w4377:dbl[][])  [unwired: 2 in]
        n2972 = Array Subset(array=w4378, index (col)=w4293) -> (w4375:dbl[][])  [unwired: 3 in]
        n2973 = Array Subset(array=w4361, index (col)=0 ("index"), length (col)=w4293) -> (w4366:dbl[][])  [unwired: 2 in]
        n2974 = Array Subset(array=w4361, index (col)=w4293) -> (w4364:dbl[][])  [unwired: 3 in]
        n2975 = for {
          tunnel: w4373 -> [w4415] mode=indexing
          tunnel: [w4414] -> w4372 mode=indexing
          workers-P: _ -> [_]
          n2976 = Reverse 1D Array(array=w4415) -> (reversed array=w4414:dbl[])
        }
        n2977 = for {
          tunnel: w4359 -> [w4411] mode=indexing
          tunnel: [w4410] -> w4358 mode=indexing
          workers-P: _ -> [_]
          n2978 = Reverse 1D Array(array=w4411) -> (reversed array=w4410:dbl[])
        }
        n2979 = for {
          tunnel: w4303 -> [w4409] mode=indexing
          tunnel: [w4408] -> w4302 mode=indexing
          workers-P: _ -> [_]
          n2980 = Reverse 1D Array(array=w4409) -> (reversed array=w4408:dbl[])
        }
        n2981 = for {
          tunnel: w4377 -> [w4417] mode=indexing
          tunnel: [w4416] -> w4376 mode=indexing
          workers-P: _ -> [_]
          n2982 = Reverse 1D Array(array=w4417) -> (reversed array=w4416:dbl[])
        }
        n2983 = for {
          tunnel: w4366 -> [w4413] mode=indexing
          tunnel: [w4412] -> w4365 mode=indexing
          workers-P: _ -> [_]
          n2984 = Reverse 1D Array(array=w4413) -> (reversed array=w4412:dbl[])
        }
        n2985 = Index Array(array=w4378, index (row)=0) -> (element=→"Waveform Graph":dbl[])  [unwired: 1 in]
        n2986 = Add(x=w4372, y=w4371) -> (x+y=w4370:dbl[][])
        n2987 = Add(x=w4358, y=w4357) -> (x+y=w4356:dbl[][])
        n2988 = Add(x=w4302, y=w4301) -> (x+y=w4286:dbl[][])
        n2989 = Add(x=w4376, y=w4375) -> (x+y=w4350:dbl[][])
        n2990 = Add(x=w4365, y=w4364) -> (x+y=w4363:dbl[][])
        n2991 = Divide(x=w4356, y=2) -> (x/y=w4354:dbl[][])
        n2992 = Divide(x=w4370, y=2) -> (x/y=w4315:dbl[][])
        n2993 = Divide(x=w4363, y=2) -> (x/y=w4317:dbl[][])
        n2994 = To Single Precision Float(number=w4350) -> (single precision float=w4349:sgl[][])
        n2995 = Transpose 2D Array(2D array=w4354) -> (transposed array=→"Data map":dbl[][])
        n2996 = To Single Precision Float(number=w4286) -> (single precision float=w4290:sgl[][])
        n2997 = To Single Precision Float(number=w4315) -> (single precision float=w4321:sgl[][])
        n2998 = To Single Precision Float(number=w4317) -> (single precision float=w4318:sgl[][])
        n2999 = call "IMAQ ArrayToImage"("Image Pixels (Float)"=w4349, "Image"=w4283) -> ("Image Out"=w4352:T2)  [unwired: 8 in, 1 out]
        n3000 = call "IMAQ ArrayToImage"("Image Pixels (Float)"=w4290, "Image"=w4282) -> ("Image Out"=w4292:T2)  [unwired: 8 in, 1 out]
        n3001 = call "IMAQ ArrayToImage"("Image Pixels (Float)"=w4321, "Image"=w4281) -> ("Image Out"=w4323:T2)  [unwired: 8 in, 1 out]
        n3002 = call "IMAQ ArrayToImage"("Image Pixels (Float)"=w4318, "Image"=w4280) -> ("Image Out"=w4320:T2)  [unwired: 8 in, 1 out]
        n3003 = call "IMAQ Symmetry"("Type of Symmetry"=w4351, "Image Src"=w4352) -> ("Image Dst Out"=w4347:T2)  [unwired: 3 in, 1 out]
        n3004 = call "IMAQ Symmetry"("Type of Symmetry"=w4291, "Image Src"=w4292) -> ("Image Dst Out"=w4288:T2)  [unwired: 3 in, 1 out]
        n3005 = call "IMAQ Symmetry"("Type of Symmetry"=w4322, "Image Src"=w4323) -> ("Image Dst Out"=→"Detection Laser X":T2)  [unwired: 3 in, 1 out]
        n3006 = call "IMAQ Symmetry"("Type of Symmetry"=w4319, "Image Src"=w4320) -> ("Image Dst Out"=→"Detection Laser Y":T2)  [unwired: 3 in, 1 out]
        n3007 = call "IMAQ Set Simple Calibration"("Calibration Axis Info"=T42 {"Origin Pixel"={"X"=0.0, "Y"=0.0}, "Angle Relative to Horizontal (deg)"=0.0, "Axis Reference"=0}, "Grid Descriptor"=T43 {"X Step"=0.3, "Y Step"=0.3, "Unit"=enum."Undefined"}, "Image"=w4347) -> ("Calibrated Image"=→"APD 1":T2)  [unwired: 7 in, 1 out]
        n3008 = call "IMAQ Set Simple Calibration"("Calibration Axis Info"=T42 {"Origin Pixel"={"X"=0.0, "Y"=0.0}, "Angle Relative to Horizontal (deg)"=0.0, "Axis Reference"=0}, "Grid Descriptor"=T43 {"X Step"=0.3, "Y Step"=0.3, "Unit"=enum."Undefined"}, "Image"=w4288) -> ("Calibrated Image"=→"APD 2":T2)  [unwired: 7 in, 1 out]
      }
    }
    n3009 = Subtract(x=w3748, y="APD 2 Offset") -> (x-y=w3745:waveform(dbl))
    n3010 = Subtract(x=w3750, y="APD 1 Offset") -> (x-y=w3746:waveform(dbl))
    n3011 = Index Array(array=w3764, index=3) -> (element=w3818:waveform(dbl))
    n3012 = Index Array(array=w3764, index=6) -> (element=w3815:waveform(dbl))
    n3013 = Build Array(w3746, w3745) -> (→"APD Chart":waveform(dbl)[])
    n3014 = Array Size(array=w3586) -> (size(s)=w3854:i32)
    n3015 = call <vilib>:"Std Deviation and Variance.vi"("X"=w3587) -> ("standard deviation"=w3757:dbl)  [unwired: 1 in, 2 out]
    n3016 = Add Array Elements(numeric array=w3587) -> (sum=w3759:u32)
    n3017 = Add Array Elements(numeric array=w3586) -> (sum=w3863:u32)
    n3018 = call <vilib>:"Std Deviation and Variance.vi"("X"=w3586) -> ("standard deviation"=w3809:dbl)  [unwired: 1 in, 2 out]
    n3019 = Divide(x="T1 offset_x (mV)", y=1000.0) -> (x/y=w3819:dbl)
    n3020 = Divide(x=w3757, y=w3756) -> (x/y=w3753:dbl)
    "Rate sigma (Hz) 2" <- w3753
    n3021 = Multiply(x=w3756, y=w3854) -> (x*y=w3758:dbl)
    "Int. Time (s)" <- w3758
    n3022 = Divide(x=w3759, y=w3758) -> (x/y=w3754:dbl)
    "APD 2 Rate (Hz)" <- w3754
    n3023 = Divide(x=w3863, y=w3758) -> (x/y=w3807:dbl)
    "APD 1 Rate (Hz)" <- w3807
    n3024 = Divide(x=w3809, y=w3756) -> (x/y=w3808:dbl)
    "Rate sigma (Hz)" <- w3808
    n3025 = Divide(x=w3753, y=w3754) -> (x/y=→"Sigma/Mean 2":dbl)